vi "15-12-13 UHR-Fleezers Control (host) - 15.2.1UCB Darwin.vi"() -> ()   [LabVIEW 2014] (continued)
        n1238 = Select(t=w1811, s="+ phase (BI DO)", f="Phase adj. (BI DO)") -> (s? t:f=w1806:i16)
        n1239 = xnode "Read/Write Control"("FPGA VI Reference In"=w1803, "Phase count adjustment (GI)"=w1841, "Phase count adjustment (GI) 2"=w1829, "Phase count adjustment (RI)"=w1822, "Phase count adjustment (Green FB)"=w1817, "Phase count adjustment (BI AO)"=w1807, "Phase count adjustment (BI D)"=w1806) -> ("FPGA VI Reference Out"=w1839:T24, "error out"=w1840:errorcluster)  [unwired: 1 in]
        n1240 = xnode "Read/Write Control"("FPGA VI Reference In"=w1839, "error in"=w1840, "+ phase (GI)"=w1837, "+ phase (GI) 2"=w1828, "+ phase (RI)"=w1823, "+ phase (Green FB)"=w1816, "+ phase (BI AO)"=w1805, "+ phase (BI D)"=w1804) -> ("error out"=w1838:errorcluster)  [unwired: 1 out]
      }
      event "Green Laser ON/OFF", "Red Laser ON/OFF", "Blue Laser ON/OFF": Value Change {
        # "This loop shouldn't be initialized.  The main 'laser ON' settings should dominate and set the others."
        n1241 = event-data() -> ()  [unwired: 7 out]
        n1242 = property on="Red Laser ON" class="Bool (strict)"("Val(Sgnl)"="Red Laser ON/OFF") -> ()  [unwired: 2 in, 2 out]
        n1243 = property on="Blue Laser ON" class="Bool (strict)"("Val(Sgnl)"="Blue Laser ON/OFF") -> ()  [unwired: 2 in, 2 out]
        n1244 = property on="Green Laser ON" class="Bool (strict)"("Val(Sgnl)"="Green Laser ON/OFF") -> ()  [unwired: 2 in, 2 out]
      }
      event "Laser interlacing mode", "Green Laser ON", "Red Laser ON", "Blue Laser ON": Value Change {
        n1245 = event-data() -> ()  [unwired: 7 out]
        n1246 = local write "Green Laser ON/OFF"("Green Laser ON") -> ()
        n1247 = local write "Blue Laser ON/OFF"("Blue Laser ON") -> ()
        n1248 = local write "Red Laser ON/OFF"("Red Laser ON") -> ()
        n1249 = case shown="True" "Green Laser ON" {
          tunnel: "Laser interlacing mode" -> [_ w1903]
          tunnel: [enum32{"Laser ON", "Laser OFF", "Interlace"}."Laser OFF" ("Green laser mode") w1903] -> w1879
          tunnel: [FALSE w1899] -> w1878
          frame False {
          }
          frame True {
            n1250 = local read "Green FB On/Off"() -> (w1900:bool)
            n1251 = Equal?(x=w1903, y=enum32{"Laser ON", "Laser OFF", "Interlace"}."Interlace") -> (x = y?=w1901:bool)
            n1252 = And(x=w1901, y=w1900) -> (x .and. y?=w1899:bool)
          }
        }
        n1253 = case shown="True" "Red Laser ON" {
          tunnel: "Laser interlacing mode" -> [_ w1896]
          tunnel: [enum32{"Laser ON", "Laser OFF", "Interlace"}."Laser OFF" ("Green laser mode") w1896] -> w1875
          tunnel: [FALSE w1892] -> w1874
          frame False {
          }
          frame True {
            n1254 = local read "Red FB On/Off"() -> (w1893:bool)
            n1255 = Equal?(x=w1896, y=enum32{"Laser ON", "Laser OFF", "Interlace"}."Interlace") -> (x = y?=w1894:bool)
            n1256 = And(x=w1894, y=w1893) -> (x .and. y?=w1892:bool)
          }
        }
        n1257 = case shown="True" "Blue Laser ON" {
          tunnel: "Laser interlacing mode" -> [_ w1887]
          tunnel: [enum32{"Laser ON", "Laser OFF", "Interlace"}."Laser OFF" ("Green laser mode") w1887] -> w1871
          tunnel: [FALSE w1885] -> w1870
          frame False {
          }
          frame True {
            n1258 = local read "Blue FB On/Off"() -> (w1886:bool)
            n1259 = Equal?(x=w1887, y=enum32{"Laser ON", "Laser OFF", "Interlace"}."Interlace") -> (x = y?=w1888:bool)
            n1260 = And(x=w1888, y=w1886) -> (x .and. y?=w1885:bool)
          }
        }
        n1261 = xnode "Read/Write Control"("FPGA VI Reference In"=w1869, "Operating Mode"=w1879, "Operating Mode 2"=w1879, "Green FB On/Off"=w1878, "Red Laser Operating Mode"=w1875, "RI Operating Mode 2"=w1875, "Red FB On/Off"=w1874, "BI Operating Mode (AO)"=w1871, "Blue Laser Operating Mode (D)"=w1871, "Blue FB On/Off"=w1870) -> ("error out"=w1880:errorcluster)  [unwired: 1 in, 1 out]
        n1262 = local read "Red FB On/Off"() -> (w1852:bool)
        n1263 = local read "Green FB On/Off"() -> (w1854:bool)
        n1264 = local read "Green Laser ON"() -> (w1853:bool)
        n1265 = local read "Red Laser ON"() -> (w1851:bool)
        n1266 = And(x=w1852, y=w1851) -> (x .and. y?=w1857:bool)
        n1267 = And(x=w1854, y=w1853) -> (x .and. y?=w1863:bool)
        n1268 = local read "Red laser intensity (V)"() -> (w1856:dbl)
        n1269 = local read "Red FB Setpoint (mV)"() -> (w1855:dbl)
        n1270 = local read "Green FB Setpoint (mV)"() -> (w1866:dbl)
        n1271 = local read "Green laser intensity (V)"() -> (w1868:dbl)
        n1272 = Multiply(x=w1856, y=1000.0) -> (x*y=w1860:dbl)
        n1273 = Subtract(x=w1855, y=5.0) -> (x-y=w1859:dbl)
        n1274 = Multiply(x=w1868, y=1000.0) -> (x*y=w1865:dbl)
        n1275 = Subtract(x=w1866, y=5.0) -> (x-y=w1864:dbl)
        n1276 = Less Or Equal?(x=w1860, y=w1859) -> (x <= y?=w1858:bool)
        n1277 = Less Or Equal?(x=w1865, y=w1864) -> (x <= y?=w1862:bool)
        n1278 = And(x=w1857, y=w1858) -> (x .and. y?=w1847:bool)
        n1279 = And(x=w1863, y=w1862) -> (x .and. y?=w1848:bool)
        n1280 = Or(x=w1848, y=w1847) -> (x .or. y?=w1846:bool)
        n1281 = case shown="True" w1846 {
          frame False {
            n1282 = local write "Laser Intensity Low (bugs to fix)"(FALSE ("Laser Intensity Low")) -> ()
          }
          frame True {
            n1283 = local write "Laser Intensity Low (bugs to fix)"(TRUE ("Laser Intensity Low")) -> ()
          }
        }
      }
      event "Invert laser interlacing": Value Change {
        n1284 = event-data() -> ()  [unwired: 7 out]
        n1285 = xnode "Read/Write Control"("FPGA VI Reference In"=w1904, "Invert GI"="Invert laser interlacing", "Invert GI 2"="Invert laser interlacing", "Invert RI"="Invert laser interlacing", "Invert RI 2"="Invert laser interlacing", "Invert BI (AO)"="Invert laser interlacing", "Invert BI (D)"="Invert laser interlacing") -> ("error out"=w1906:errorcluster)  [unwired: 1 in, 1 out]
      }
      event "Green FB Setpoint (mV)", "Green FB Gains", "Green FB On/Off", "Green Intensity % (FB OFF)", "Green int current ON count adj": Value Change {
        n1286 = event-data() -> ()  [unwired: 7 out]
        n1287 = local read "Green FB Setpoint (mV)"() -> (w1926:dbl)
        n1288 = Multiply(x=w1926, y=3.2767) -> (x*y=w1925:dbl)
        n1289 = local read "Green Intensity % (FB OFF)"() -> (w1929:dbl)
        n1290 = Multiply(x=w1929, y=655.35) -> (x*y=w1930:dbl)
        n1291 = To Unsigned Word Integer(number=w1930) -> (unsigned 16bit integer=w1928:u16)
        n1292 = local read "Green int current ON count adj"() -> (w1932:u32)
        n1293 = local read "Laser interlacing mode"() -> (w1923:enum32{"Laser ON", "Laser OFF", "Interlace"})
        n1294 = local read "Green FB Gains"() -> (w1920:T11)
        n1295 = local read "Green Laser ON"() -> (w1924:bool)
        n1296 = local read "Green FB On/Off"() -> (w1933:bool)
        n1297 = Equal?(x=w1923, y=enum32{"Laser ON", "Laser OFF", "Interlace"}."Interlace") -> (x = y?=w1921:bool)
        n1298 = Unbundle By Name(w1920) -> ("proportional gain (Kc)"=w1919:i16, "integral gain (Kc*Ts/Ti)"=w1918:i16, "derivative gain (Kc*Td/Ts)"=w1917:i16)
        n1299 = Compound Arithmetic op=AND(w1921, w1933, w1924) -> (w1907:bool)
        n1300 = local read "Green FB Setpoint (mV)"() -> (w1911:dbl)
        n1301 = local read "Green laser intensity (V)"() -> (w1914:dbl)
        n1302 = xnode "Read/Write Control"("FPGA VI Reference In"=w1916, "Green FB Setpoint"=w1925, "Green FB On/Off"=w1907, "Current Out"=w1928, "Green int current ON count adj"=w1932, "P3"=w1919, "I3"=w1918, "D3"=w1917) -> ("error out"=w1934:errorcluster)  [unwired: 1 in, 1 out]
        n1303 = Multiply(x=w1914, y=1000.0) -> (x*y=w1910:dbl)
        n1304 = Subtract(x=w1911, y=5.0) -> (x-y=w1909:dbl)
        n1305 = Less Or Equal?(x=w1910, y=w1909) -> (x <= y?=w1908:bool)
        n1306 = And(x=w1907, y=w1908) -> (x .and. y?=w1915:bool)
        n1307 = case shown="True" w1915 {
          frame False {
            n1308 = local write "Laser Intensity Low (bugs to fix)"(FALSE ("Laser Intensity Low")) -> ()
          }
          frame True {
            n1309 = local write "Laser Intensity Low (bugs to fix)"(TRUE ("Laser Intensity Low")) -> ()
          }
        }
      }
      event "Blue FB Setpoint (mV)", "Blue FB Gains", "Blue FB On/Off", "Blue Intensity % (FB OFF)", "Blue int AO ON count adjust": Value Change {
        # "Triggers blue laser serial command"
        # "16 bit analog out"
        n1310 = event-data() -> ()  [unwired: 7 out]
        n1311 = Multiply(x="Blue FB Setpoint (mV)", y=3.2767) -> (x*y=w1954:dbl)
        n1312 = Multiply(x="Blue Intensity % (FB OFF)", y=0.8) -> (x*y=w1937:dbl)
        n1313 = Number To Decimal String(number=w1937) -> (decimal integer string=w1938:string)  [unwired: 1 in]
        n1314 = Multiply(x="Blue Intensity % (FB OFF)", y=655.35) -> (x*y=w1957:dbl)
        n1315 = local write "Blue Laser Power (mW)\n(Constant Power Mode)"(w1938) -> ()
        n1316 = To Unsigned Word Integer(number=w1957) -> (unsigned 16bit integer=w1956:u16)
        n1317 = local read "Laser interlacing mode"() -> (w1952:enum32{"Laser ON", "Laser OFF", "Interlace"})
        n1318 = Unbundle By Name("Blue FB Gains") -> ("proportional gain (Kc)"=w1949:i16, "integral gain (Kc*Ts/Ti)"=w1948:i16, "derivative gain (Kc*Td/Ts)"=w1947:i16)
        n1319 = local read "Blue Laser ON"() -> (w1942:bool)
        n1320 = Equal?(x=w1952, y=enum32{"Laser ON", "Laser OFF", "Interlace"}."Interlace") -> (x = y?=w1950:bool)
        n1321 = Compound Arithmetic op=AND(w1950, "Blue FB On/Off", w1942) -> (w1953:bool)
        n1322 = xnode "Read/Write Control"("FPGA VI Reference In"=w1941, "Blue FB Setpoint"=w1954, "Blue FB On/Off"=w1953, "BI Current Out"=w1956, "Blue current ON count adj (AO)"="Blue int AO ON count adjust", "P5"=w1949, "I5"=w1948, "D5"=w1947) -> ("error out"=w1959:errorcluster)  [unwired: 1 in, 1 out]
      }
      event "Red FB Setpoint (mV)", "Red FB Gains", "Red FB On/Off", "Red Intensity % (FB OFF)": Value Change {
        n1323 = event-data() -> ()  [unwired: 7 out]
        n1324 = local read "Red FB Setpoint (mV)"() -> (w1980:dbl)
        n1325 = Multiply(x=w1980, y=3.2767) -> (x*y=w1979:dbl)
        n1326 = local read "Red Intensity % (FB OFF)"() -> (w1970:dbl)
        n1327 = Multiply(x=w1970, y=655.35) -> (x*y=w1983:dbl)
        n1328 = To Unsigned Word Integer(number=w1983) -> (unsigned 16bit integer=w1982:u16)
        n1329 = local read "Laser interlacing mode"() -> (w1977:enum32{"Laser ON", "Laser OFF", "Interlace"})
        n1330 = local read "Red FB Gains"() -> (w1974:T11)
        n1331 = local read "Red Laser ON"() -> (w1978:bool)
        n1332 = local read "Red FB On/Off"() -> (w1985:bool)
        n1333 = Equal?(x=w1977, y=enum32{"Laser ON", "Laser OFF", "Interlace"}."Interlace") -> (x = y?=w1975:bool)
        n1334 = Unbundle By Name(w1974) -> ("proportional gain (Kc)"=w1973:i16, "integral gain (Kc*Ts/Ti)"=w1972:i16, "derivative gain (Kc*Td/Ts)"=w1971:i16)
        n1335 = Compound Arithmetic op=AND(w1975, w1985, w1978) -> (w1962:bool)
        n1336 = local read "Red laser intensity (V)"() -> (w1961:dbl)
        n1337 = local read "Red FB Setpoint (mV)"() -> (w1960:dbl)
        n1338 = xnode "Read/Write Control"("FPGA VI Reference In"=w1969, "Red FB Setpoint"=w1979, "Red FB On/Off"=w1962, "RI Current Out"=w1982, "P4"=w1973, "I4"=w1972, "D4"=w1971) -> ("error out"=w1986:errorcluster)  [unwired: 1 in, 1 out]
        n1339 = Multiply(x=w1961, y=1000.0) -> (x*y=w1966:dbl)
        n1340 = Subtract(x=w1960, y=5.0) -> (x-y=w1965:dbl)
        n1341 = Less Or Equal?(x=w1966, y=w1965) -> (x <= y?=w1964:bool)
        n1342 = And(x=w1962, y=w1964) -> (x .and. y?=w1963:bool)
        n1343 = case shown="False" w1963 {
          frame False {
            n1344 = local write "Laser Intensity Low (bugs to fix)"(FALSE ("Laser Intensity Low")) -> ()
          }
          frame True {
            n1345 = local write "Laser Intensity Low (bugs to fix)"(TRUE ("Laser Intensity Low")) -> ()
          }
        }
      }
      event "+ phase (APD 1 Gate)", "- phase (APD 1 Gate)", "+ phase (APD 2 Gate)", "- phase (APD 2 Gate)", "+ phase (APD 3 Gate)", "- phase (APD 3 Gate)", "+ phase (APD Acq)", "- phase (APD Acq)": Value Change {
        n1346 = event-data() -> ()  [unwired: 7 out]
        n1347 = local read "Phase Adj. (APD 1 Gate)"() -> (w2009:i16)
        n1348 = Or(x="- phase (APD 1 Gate)", y="+ phase (APD 1 Gate)") -> (x .or. y?=w2011:bool)
        n1349 = Negate(x=w2009) -> (-x=w2016:i16)
        n1350 = Select(t=w2016, s="+ phase (APD 1 Gate)", f=w2009) -> (s? t:f=w2015:i16)
        n1351 = local read "Phase Adj. (APD 2 Gate)"() -> (w2006:i16)
        n1352 = Or(x="- phase (APD 2 Gate)", y="+ phase (APD 2 Gate)") -> (x .or. y?=w2004:bool)
        n1353 = Negate(x=w2006) -> (-x=w2008:i16)
        n1354 = Select(t=w2008, s="+ phase (APD 2 Gate)", f=w2006) -> (s? t:f=w2005:i16)
        n1355 = Negate(x="Phase Adj. (APD 3 Gate)") -> (-x=w2003:i16)
        n1356 = Or(x="- phase (APD 3 Gate)", y="+ phase (APD 3 Gate)") -> (x .or. y?=w1999:bool)
        n1357 = Select(t=w2003, s="+ phase (APD 3 Gate)", f="Phase Adj. (APD 3 Gate)") -> (s? t:f=w2000:i16)
        n1358 = local read "Phase Adj. (APD Acq)"() -> (w1997:i16)
        n1359 = Or(x="- phase (APD Acq)", y="+ phase (APD Acq)") -> (x .or. y?=w1995:bool)
        n1360 = Negate(x=w1997) -> (-x=w1998:i16)
        n1361 = Select(t=w1998, s="+ phase (APD Acq)", f=w1997) -> (s? t:f=w1996:i16)
        n1362 = xnode "Read/Write Control"("FPGA VI Reference In"=w1989, "Phase count adjustment (APD 1 Gate)"=w2015, "Phase count adjustment (APD 2 Gate)"=w2005, "Phase count adjustment (APD 3 Gate)"=w2000, "Phase Count Adjustment (APD Acq)"=w1996) -> ("FPGA VI Reference Out"=w2013:T24, "error out"=w2014:errorcluster)  [unwired: 1 in]
        n1363 = xnode "Read/Write Control"("FPGA VI Reference In"=w2013, "error in"=w2014, "+ phase (APD 1 Gate)"=w2011, "+ phase (APD 2 Gate)"=w2004, "+ phase (APD 3 Gate)"=w1999, "+ phase (APD Acq)"=w1995) -> ("error out"=w2012:errorcluster)  [unwired: 1 out]
      }
      event "Invert APD Gate", "APD Gate ON Count", "APD Gate OFF Count", "APD Gate", "APD Integration Time (s)", "APD AO Scale Factor", "Duty Frequency (ON 1/N cycles)", "Interlace ON count", "Interlace OFF count": Value Change {
        n1364 = event-data() -> ()  [unwired: 7 out]
        n1365 = Add(x="Interlace ON count", y="Interlace OFF count") -> (x+y=w2023:u16)
        n1366 = Add(x="APD Gate ON Count", y="APD Gate OFF Count") -> (x+y=w2034:u16)
        n1367 = Multiply(x="Duty Frequency (ON 1/N cycles)", y=w2023) -> (x*y=w2019:u16)
        "Green AI Count" <- w2019
        "Red AI Count" <- w2019
        "Blue AI Count" <- w2019
        n1368 = Subtract(x=w2019, y="Interlace ON count") -> (x-y=w2022:u16)
        n1369 = Multiply(x=w2034, y="Duty Frequency (ON 1/N cycles)") -> (x*y=w2033:u16)
        n1370 = Subtract(x=w2033, y="APD Gate ON Count") -> (x-y=w2032:u16)
        n1371 = local read "DMA Update Period (s)"() -> (w2035:dbl)
        n1372 = Multiply(x="APD Integration Time (s)", y=40000000.0) -> (x*y=w2039:dbl)
        n1373 = Reciprocal(x="APD Integration Time (s)") -> (1/x=→"APD Acq Rate (Hz)":dbl)
        n1374 = To Unsigned Long Integer(number=w2039) -> (unsigned 32bit integer=w2025:u32)
        "APD Int. Count" <- w2025
        n1375 = local read "Number of APDs"() -> (w2018:u8)
        n1376 = Divide(x=w2035, y="APD Integration Time (s)") -> (x/y=w2037:dbl)
        n1377 = Multiply(x=w2018, y=w2037) -> (x*y=w2036:dbl)
        n1378 = local write "APD Samples/FIFO Acq."(w2037) -> ()
        n1379 = local write "APD Elements/DMA read"(w2036) -> ()
        n1380 = xnode "Read/Write Control"("FPGA VI Reference In"=w2017, "Invert APD Gate"="Invert APD Gate", "APD Gate ON Count"="APD Gate ON Count", "APD Gate OFF Count"=w2032, "APD Acq Rate Count"=w2025, "APD Gate Operating Mode"="APD Gate", "APD AO scale factor"="APD AO Scale Factor", "Green interlace ON count"="Interlace ON count", "Green interlace OFF count"=w2022, "Green interlace ON count 2"="Interlace ON count", "Green interlace OFF count 2"=w2022, "Green FB Count"=w2019, "Red interlace ON count"="Interlace ON count", "Red interlace OFF count"="Interlace OFF count", "Blue ON count (AO)"="Interlace ON count", "Blue OFF count (AO)"="Interlace OFF count", "Blue interlace OFF count (D)"="Interlace OFF count", "Blue interlace ON count (D)"="Interlace ON count") -> ("error out"=w2041:errorcluster)  [unwired: 1 in, 1 out]
      }
      event "Neg. TTrig FPGA": Value Change {
        n1381 = event-data() -> ()  [unwired: 7 out]
        n1382 = xnode "Read/Write Control"("FPGA VI Reference In"=w2042, "TTrig Negate Pos"="Neg. TTrig FPGA") -> ()  [unwired: 1 in, 2 out]
      }
      event "Test ttrig": Value Change {
        n1383 = event-data() -> ()  [unwired: 7 out]
        n1384 = xnode "Read/Write Control"("FPGA VI Reference In"=w2044, "TTrig?"=TRUE) -> ("error out"=w2046:errorcluster)  [unwired: 1 in, 1 out]
      }
      event "Number of F/B Scans (AOD)", "Scan Speed (nm/s)", "Scan BD", "Initial delta (MHz)", "Step Size (nm)", "Scan Range (nm)": Value Change {
        w2110 = 123.0  # AOM cal (nm/MHz)
        n1385 = event-data() -> ()  [unwired: 7 out]
        n1386 = local read "BD 1 Frequency 1 (MHz)"() -> (w2093:dbl)
        n1387 = local read "AOM X Cal (nm/MHz)"() -> (w2085:dbl)
        n1388 = local read "X RF Frequency Limits (MHz)"() -> (w2097:T18)
        n1389 = local read "Y RF Frequency Limits (MHz)"() -> (w2094:T18)
        n1390 = local read "BD 2 Frequency 1 (MHz)"() -> (w2099:dbl)
        n1391 = Negate(x="Scan Range (nm)") -> (-x=w2063:dbl)
        n1392 = Divide(x=w2063, y=w2085) -> (x/y=w2067:dbl)
        n1393 = Select(t=w2097, s="Scan BD", f=w2094) -> (s? t:f=w2096:T18)
        n1394 = Select(t=w2093, s="Scan BD", f=w2099) -> (s? t:f=w2098:dbl)
        n1395 = Unbundle By Name(w2096) -> ("Maximum"=w2105:dbl, "Minimum"=w2104:dbl)
        n1396 = Add(x=w2067, y=w2098) -> (x+y=w2102:dbl)
        n1397 = Divide(x=w2063, y="Step Size (nm)") -> (x/y=w2082:dbl)
        n1398 = Divide(x="Step Size (nm)", y=w2085) -> (x/y=w2091:dbl)
        n1399 = Absolute Value(x=w2082) -> (abs(x)=w2066:dbl)
        n1400 = Sign(1:w2063) -> (0:w2064:dbl)
        n1401 = In Range and Coerce(upper limit=w2105, x=w2102, lower limit=w2104) -> (coerced(x)=w2101:dbl, In Range?=w2103:bool)
        n1402 = To Unsigned Quad Integer(1:w2066) -> (0:w2081:u64)
        "Scan steps (AOD)" <- w2081
        n1403 = call "IR AOM freq to word.vi"("Frequency In (MHz)"=w2091) -> ("Frequency Word Out (double)"=w2088:dbl)
        n1404 = Multiply(x=w2064, y=w2088) -> (x*y=w2065:dbl)
        n1405 = Subtract(x=w2102, y=w2101) -> (x-y=w2100:dbl)
        n1406 = To Quad Integer(1:w2065) -> (0:w2087:i64)
        "Incr. int (AOD)" <- w2087
        n1407 = Subtract(x=w2067, y=w2100) -> (x-y=w2086:dbl)
        "Scan Range (MHz)" <- w2086
        n1408 = Select(t=w2067, s=w2103, f=w2086) -> (s? t:f=w2106:dbl)
        n1409 = Multiply(x=w2086, y=w2085) -> (x*y=w2084:dbl)
        n1410 = Decrement(x=w2081) -> (x-1=w2134:u64)
        n1411 = Negate(x=w2084) -> (-x=w2080:dbl)
        n1412 = local write "Scan Range (nm)"(w2080) -> ()
        n1413 = Divide(x=w2106, y=w2134) -> (x/y=w2090:dbl)
        "Scan Increment (MHz)" <- w2090
        n1414 = call "IR AOM freq to word.vi"("Frequency In (MHz)"=w2090) -> ("Frequency Word Out (double)"=w2089:dbl)
        n1415 = Divide(x="Step Size (nm)", y="Scan Speed (nm/s)") -> (x/y=w2077:dbl)
        n1416 = To Quad Integer(1:w2089) -> ()  [unwired: 1 out]
        n1417 = local read "Number Interlace Sets"() -> (w2061:u8)
        n1418 = local read "AI Count (ticks)"() -> (w2062:u16)
        n1419 = local read "Total Counts (ticks)"() -> (w2060:u16)
        n1420 = local read "# Samples/trap"() -> (w2092:u32)
        n1421 = Multiply(x=w2062, y=w2061) -> (x*y=w2059:u16)
        n1422 = Divide(x=w2060, y=w2059) -> (x/y=w2058:dbl)
        n1423 = Select(t=w2093, s="Scan BD", f=w2099) -> (s? t:f=w2131:dbl)
        "Initial freq. (MHz)" <- w2131
        n1424 = Add(x=w2106, y=w2131) -> (x+y=→"Final freq. (MHz)":dbl)
        n1425 = Divide(x=w2060, y=40000000.0) -> (x/y=w2076:dbl)
        n1426 = Divide(x=w2077, y=w2076) -> (x/y=w2075:dbl)
        n1427 = To Unsigned Quad Integer(1:w2075) -> (0:w2050:u64)
        n1428 = Quotient & Remainder(x=w2050, y=u64 2) -> (x-y*floor(x/y)=w2054:u64)  [unwired: 1 out]
        n1429 = Equal?(x=w2054, y=u64 0) -> (x = y?=w2052:bool)
        n1430 = Decrement(x=w2050) -> (x-1=w2051:u64)
        n1431 = Select(t=w2050, s=w2052, f=w2051) -> (s? t:f=w2049:u64)
        "Cycles/step (AOD)" <- w2049
        n1432 = xnode "Read/Write Control"("FPGA VI Reference In"=w2048, "Scan steps"=w2081, "Number of scans"="Number of F/B Scans (AOD)", "Cycles per step"=w2049, "Scan freq.  increment"=w2087, "Scan BD"="Scan BD") -> ("error out"=w2140:errorcluster)  [unwired: 1 in, 1 out]
        n1433 = Multiply(x=w2081, y=w2049) -> (x*y=w2135:u64)
        n1434 = Multiply(x=w2135, y=u64 2) -> (x*y=w2057:u64)
        n1435 = Multiply(x=w2058, y=w2057) -> (x*y=w2056:dbl)
        "Data points/scan (f/b)" <- w2056
        n1436 = Multiply(x=w2056, y="Number of F/B Scans (AOD)") -> (x*y=w2138:dbl)
        "Data points/scans" <- w2138
        n1437 = Divide(x=w2138, y=w2092) -> (x/y=→"N sets should be saved":dbl)
        n1438 = Multiply(x=w2135, y=w2076) -> (x*y=w2074:dbl)
        "Time/Scan (s) (AOD)" <- w2074
        n1439 = Select(t=w2106, s="Scan BD", f=0.0) -> (s? t:f=w2132:dbl)
        n1440 = Select(t=0.0, s="Scan BD", f=w2106) -> (s? t:f=w2128:dbl)
        n1441 = local read "BD 2 Frequency 2 (MHz)"() -> (w2124:dbl)
        n1442 = local read "BD 1 Frequency 2 (MHz)"() -> (w2127:dbl)
        n1443 = Add(x=w2128, y=w2099) -> (x+y=w2125:dbl)
        n1444 = Add(x=w2093, y=w2132) -> (x+y=w2126:dbl)
        n1445 = Multiply(x=w2074, y=2.0) -> (x*y=w2073:dbl)
        n1446 = Multiply(x=w2073, y="Number of F/B Scans (AOD)") -> (x*y=w2070:dbl)
        n1447 = Divide(x=w2070, y=60.0) -> (x/y=→"Time to Finish All (min)":dbl)
        n1448 = Add(x="Trap 2 Bead Size (nm)", y="Trap 1 Bead Size (nm)") -> (x+y=w2114:dbl)
        n1449 = Divide(x=w2114, y=2.0) -> (x/y=w2108:dbl)
        n1450 = local read "Initial delta (MHz)"() -> (w2111:dbl)
        n1451 = Subtract(x=w2125, y=w2124) -> (x-y=w2122:dbl)
        n1452 = Subtract(x=w2126, y=w2127) -> (x-y=w2123:dbl)
        n1453 = Square(x=w2122) -> (x^2=w2121:dbl)
        n1454 = Square(x=w2123) -> (x^2=w2120:dbl)
        n1455 = Add(x=w2120, y=w2121) -> (x+y=w2119:dbl)
        n1456 = Square Root(x=w2119) -> (sqrt(x)=w2118:dbl)
        "Final delta (MHz)" <- w2118
        n1457 = Multiply(x=w2110, y=w2118) -> (x*y=w2117:dbl)
        n1458 = Multiply(x=w2111, y=w2110) -> (x*y=w2109:dbl)
        n1459 = Subtract(x=w2109, y=w2108) -> (x-y=→"Initial sep (nm)":dbl)
        n1460 = Subtract(x=w2117, y=w2108) -> (x-y=→"Final sep (nm)":dbl)
      }
      event "Freq or Amp switch first", "Swap F1 and F2", "Freq switch delay", "Amp switch delay": Value Change {
        n1461 = event-data() -> ()  [unwired: 7 out]
        n1462 = local read "Amp switch delay"() -> (w2142:u16)
        n1463 = local read "Swap F1 and F2"() -> (w2143:bool)
        n1464 = xnode "Read/Write Control"("FPGA VI Reference In"=w2141, "Swap F1 and F2"=w2143, "Amp switch delay"=w2142) -> ("error out"=w2144:errorcluster)  [unwired: 1 in, 1 out]
      }
      event "Scan steps (MCL)", "Number of scans (MCL)", "Scan Range (V)\n(of steps)", "2D or 1D Scan", "N APD Samp/step", "Fast Scan Dir", "Continuous MCL Scanning", "Scan lines (y)": Value Change {
        w2147 = 32767.0 ("y")
        n1465 = event-data() -> ()  [unwired: 7 out]
        n1466 = Select(t="Scan lines (y)", s="2D or 1D Scan", f="Number of scans (MCL)") -> (s? t:f=w2152:u64)
        n1467 = Decrement(x="Scan steps (MCL)") -> (x-1=w2168:u64)
        n1468 = Divide(x="Scan Range (V)\n(of steps)", y=w2168) -> (x/y=w2167:dbl)
        "Desired Scan Incr (V)" <- w2167
        n1469 = local read "APD Integration Time (s)"() -> (w2160:dbl)
        n1470 = Multiply(x=w2167, y=w2147) -> (x*y=w2176:dbl)
        n1471 = Divide(x=w2176, y=10.0) -> (x/y=w2166:dbl)
        "Desired incr (int)" <- w2166
        n1472 = local read "Update Count (MCL)"() -> (w2172:u32)
        n1473 = Round Toward -Infinity(1:w2166) -> (0:w2175:dbl)
        n1474 = To Word Integer(number=w2175) -> (16bit integer=w2150:i16)
        "Actual Incr. int (MCL)" <- w2150
        n1475 = Multiply(x=w2160, y=40000000.0) -> (x*y=w2173:dbl)
        n1476 = Divide(x=w2173, y=w2172) -> (x/y=w2171:dbl)
        n1477 = Multiply(x=i16 10, y=w2150) -> (x*y=w2148:i16)
        n1478 = Multiply(x="N APD Samp/step", y=w2171) -> (x*y=w2170:dbl)
        "Cycles/step (MCL)" <- w2170
        n1479 = Divide(x=w2148, y=w2147) -> (x/y=→"Actual MCL Inc (V)":dbl)
        n1480 = Multiply(x="N APD Samp/step", y="Scan steps (MCL)") -> (x*y=w2162:dbl)
        n1481 = local read "APD Samples/FIFO Acq."() -> (w2159:dbl)
        n1482 = Multiply(x=w2162, y=u64 2) -> (x*y=w2161:dbl)
        "Data points/scan (f+b)" <- w2161
        n1483 = Multiply(x=w2161, y=w2152) -> (x*y=w2179:dbl)
        "Data points/scans (MCL)" <- w2179
        n1484 = Multiply(x=w2160, y=w2161) -> (x*y=w2153:dbl)
        "Time/f+b scan (s) (MCL)" <- w2153
        n1485 = Divide(x=w2179, y=w2159) -> (x/y=→"N sets should be saved (MCL)":dbl)
        n1486 = Multiply(x=w2153, y=w2152) -> (x*y=→"Total Time (s)":dbl)
        n1487 = Not(x="Fast Scan Dir") -> (.not. x?=w2157:bool)
        n1488 = xnode "Read/Write Control"("FPGA VI Reference In"=w2145, "Scan steps (MCL)"="Scan steps (MCL)", "Number of scans (MCL)"=w2152, "Cycles per step (MCL)"=w2170, "Scan freq.  increment (MCL)"=w2150, "1D or 2D Scan?"="2D or 1D Scan", "MCL Scan Axis"=w2157, "Cont. Scan (MCL)"="Continuous MCL Scanning") -> ("error out"=w2181:errorcluster)  [unwired: 1 in, 1 out]
      }
      event "Read Cal": Value Change {
        w2193 = 1000.0 ("y")
        n1489 = event-data() -> ()  [unwired: 7 out]
        n1490 = local read "Save file name"() -> (w2212:path)
        n1491 = local write "Read Cal"(FALSE ("Read Cal")) -> ()
        n1492 = Strip Path(path=w2212) -> (stripped path=w2211:path)  [unwired: 1 out]
        n1493 = Path To String(path=w2211) -> (string=w2210:string)
        n1494 = Concatenate Strings(w2210, "\\current.cal" ("string")) -> (w2208:string)
        n1495 = String To Path(string=w2208) -> (path=w2207:path)
        n1496 = Open/Create/Replace File(file path (use dialog)=w2207, operation (0:open)=T33."open", access (0:read/write)=enum16{"read/write", "read-only", "write-only"}."read-only") -> (refnum out=w2215:refnum<file>, error out=w2201:errorcluster)  [unwired: 1 in, 3 out]
        n1497 = Deny Access(4:w2201, 7:w2215) -> (0:w2200:errorcluster, 3:w2206:refnum<file>)  [unwired: 1 out]
        n1498 = Read from Binary File(5:0.0, 8:w2200, 9:T32."big-endian, network order" ("byte order (0:big-endian, network order)"), 10:-1 ("count (1)"), 11:w2206) -> (0:w2199:errorcluster, 2:w2197:dbl[], 3:w2202:refnum<file>)  [unwired: 2 out]
        n1499 = Array To Cluster(array=w2197) -> (cluster=w2196:T35)
        n1500 = Unbundle(w2196) -> ("[0]"=w2190:dbl, "[1]"=w2184:dbl, "[2]"=w2188:dbl, "[3]"=w2182:dbl, "[4]"=w2195:dbl, "[5]"=w2194:dbl)
        n1501 = Close File(refnum=w2202, error in=w2199) -> (error out=→"Read cal error":errorcluster)  [unwired: 1 out]
        n1502 = Multiply(x=w2195, y=w2193) -> (x*y=w2189:dbl)
        n1503 = Multiply(x=w2194, y=w2193) -> (x*y=w2183:dbl)
        n1504 = Bundle By Name(cluster="T1 calibration", "T1 alpha_x (nm/V)"=w2190, "T1 offset_x (mV)"=w2189, "T1 kappa_x (pN/nm)"=w2188) -> (w2187:T6)
        n1505 = Bundle By Name(cluster="T2 calibration", "T2 alpha_x (nm/V)"=w2184, "T2 offset_x (mV)"=w2183, "T2 kappa_x (pN/nm)"=w2182) -> (w2185:T5)
        n1506 = local write "T1 calibration"(w2187) -> ()
        n1507 = local write "T2 calibration"(w2185) -> ()
      }
      event "Abort MCL Scan": Value Change {
        n1508 = event-data() -> ()  [unwired: 7 out]
        n1509 = local write "MCL Scanning"(FALSE ("MCL Scanning")) -> ()
        n1510 = xnode "Read/Write Control"("FPGA VI Reference In"=w2216, "Abort scan (MCL)"="Abort MCL Scan") -> ("error out"=w2219:errorcluster)  [unwired: 1 in, 1 out]
      }
      event "Update Count (MCL)": Value Change {
        n1511 = event-data() -> ()  [unwired: 7 out]
        n1512 = xnode "Read/Write Control"("FPGA VI Reference In"=w2220, "MCL count"="Update Count (MCL)") -> ("error out"=w2222:errorcluster)  [unwired: 1 in, 1 out]
      }
      event "+ phase (MCL)", "- phase (MCL)": Value Change {
        n1513 = event-data() -> ()  [unwired: 7 out]
        n1514 = Or(x="- phase (MCL)", y="+ phase (MCL)") -> (x .or. y?=w2226:bool)
        n1515 = Negate(x="Phase adjust (MCL)") -> (-x=w2232:i16)
        n1516 = Select(t=w2232, s="+ phase (MCL)", f="Phase adjust (MCL)") -> (s? t:f=w2230:i16)
        n1517 = xnode "Read/Write Control"("FPGA VI Reference In"=w2223, "Phase count adjustment (MCL)"=w2230) -> ("FPGA VI Reference Out"=w2227:T24, "error out"=w2228:errorcluster)  [unwired: 1 in]
        n1518 = xnode "Read/Write Control"("FPGA VI Reference In"=w2227, "error in"=w2228, "+ phase (MCL)"=w2226) -> ("error out"=w2225:errorcluster)  [unwired: 1 out]
      }
      event "Abort AOD Scan": Value Change {
        n1519 = event-data() -> ()  [unwired: 7 out]
        n1520 = xnode "Read/Write Control"("FPGA VI Reference In"=w2233, "Abort scan"="Abort AOD Scan") -> ("error out"=w2235:errorcluster)  [unwired: 1 in, 1 out]
      }
      event "Continuous AOD Scanning": Value Change {
        n1521 = event-data() -> ()  [unwired: 7 out]
        n1522 = xnode "Read/Write Control"("FPGA VI Reference In"=w2236, "Cont. Scan"="Continuous AOD Scanning") -> ("error out"=w2238:errorcluster)  [unwired: 1 in, 1 out]
      }
      event "Index": Value Change {
        n1523 = event-data() -> ()  [unwired: 7 out]
        n1524 = call "Create new save file.vi"("Insert"="", "Ext"=".dat" ("string"), "Index In"="Index") -> ("Path Out"=→"Save file name":path, "Index Out"=w2239:dbl)
        "Save index" <- w2239
        n1525 = local write "Index"(w2239) -> ()
      }
      event "AO1", "AO2": Value Change {
        w2253 = 10.0 ("y")
        w2252 = 32767.0 ("y")
        n1526 = event-data() -> ()  [unwired: 7 out]
        n1527 = local read "AO2"() -> (w2251:dbl)
        n1528 = local read "AO1"() -> (w2248:dbl)
        n1529 = Multiply(x=w2248, y=w2252) -> (x*y=w2247:dbl)
        n1530 = Multiply(x=w2251, y=w2252) -> (x*y=w2250:dbl)
        n1531 = Divide(x=w2247, y=w2253) -> (x/y=w2246:dbl)
        n1532 = Divide(x=w2250, y=w2253) -> (x/y=w2249:dbl)
        n1533 = To Word Integer(number=w2246) -> (16bit integer=w2254:i16)
        n1534 = To Word Integer(number=w2249) -> (16bit integer=w2255:i16)
        n1535 = xnode "Read/Write Control"("FPGA VI Reference In"=w2244, "AO1"=w2254, "AO2"=w2255) -> ("error out"=w2245:errorcluster)  [unwired: 1 in, 1 out]
      }
      event "Inject Pump 1": Value Change {
        n1536 = event-data() -> ()  [unwired: 7 out]
        n1537 = local read "Use Harvard pumps\nfor beads (else Chemyx)"() -> (w2257:bool)
        n1538 = case shown="True" w2257 {
          tunnel: "Inject Pump 1" -> [w2261 w2302]
          tunnel: w2256 -> [_ w2303]
          frame False {
            n1539 = local read "Pump write delay (ms)"() -> (w2260:dbl)
            n1540 = local read "Chemyx Syringe Pump Serial Port"() -> (w2259:refnum<visa-resource-name>)
            n1541 = case shown="True" w2261 {
              tunnel: w2260 -> [w2267 w2281]
              tunnel: w2259 -> [w2264 w2280]
              frame False {
                n1542 = flat-sequence {
                  tunnel: w2264 -> [w2268]
                  tunnel: [w2268] -> w2265
                  tunnel: w2267 -> [_]
                  tunnel: [w2271] -> w2266
                  tunnel: w2265 -> [w2271]
                  tunnel: w2266 -> [w2272]
                  tunnel: [w2272] -> w2262
                  tunnel: [w2274] -> w2263
                  tunnel: w2262 -> [w2274]
                  tunnel: w2263 -> [w2276]
                  frame #0 {
                    n1543 = call "Write to pump.vi"("string"="enter pump1", "VISA resource name"=w2268) -> ()  [unwired: 1 out]
                  }
                  frame #1 {
                    n1544 = Wait (ms)(milliseconds to wait="Pump pause delay (ms)") -> ()  [unwired: 1 out]
                  }
                  frame #2 {
                    n1545 = call "Write to pump.vi"("string"="stop", "VISA resource name"=w2272) -> ()  [unwired: 1 out]
                  }
                  frame #3 {
                    n1546 = Wait (ms)(milliseconds to wait=u32 500) -> ()  [unwired: 1 out]
                  }
                  frame #4 {
                    n1547 = call "Write to pump.vi"("string"="stop", "VISA resource name"=w2276) -> ()  [unwired: 1 out]
                  }
                }
              }
              frame True {
                n1548 = flat-sequence {
                  tunnel: w2280 -> [w2290]
                  tunnel: w2281 -> [w2285]
                  tunnel: w2281 -> [w2292]
                  tunnel: w2280 -> [w2293]
                  tunnel: [w2293] -> w2278
                  tunnel: [w2295] -> w2279
                  tunnel: w2278 -> [w2295]
                  tunnel: w2279 -> [w2297]
                  frame #0 {
                    n1549 = local read "All Pump Parameters"() -> (w2284:T7)
                    n1550 = Unbundle By Name(w2284) -> ("Pump 1"=w2291:T36)
                    n1551 = call "Set pump parameters.vi"("Pump write delay (ms)"=w2285, "Volume (uL)"="Ch 1 Inject Volume (uL)", "Rate (uL/h)"="Ch 1 Inject Rate (ul/h)", "Units"=4.0, "Pump #"=1.0, "Pump Parameters In"=w2291, "VISA resource name"=w2290) -> ("Pump Parameters Out"=w2283:T36)  [unwired: 3 in]
                    n1552 = Bundle By Name(cluster=w2284, "Pump 1"=w2283) -> (w2282:T7)
                    n1553 = local write "All Pump Parameters"(w2282) -> ()
                  }
                  frame #1 {
                    n1554 = Wait (ms)(milliseconds to wait=w2292) -> ()  [unwired: 1 out]
                  }
                  frame #2 {
                    n1555 = call "Write to pump.vi"("string"="start", "VISA resource name"=w2293) -> ()  [unwired: 1 out]
                  }
                  frame #3 {
                    n1556 = Wait (ms)(milliseconds to wait=u32 500) -> ()  [unwired: 1 out]
                  }
                  frame #4 {
                    n1557 = call "Write to pump.vi"("string"="start", "VISA resource name"=w2297) -> ()  [unwired: 1 out]
                  }
                }
              }
            }
          }
          frame True {
            n1558 = case shown="False" w2302 {
              tunnel: w2303 -> [w2315 w2325]
              frame False {
                n1559 = flat-sequence {
                  tunnel: w2315 -> [w2317]
                  frame #0 {
                    n1560 = local write "Flushing P1"(FALSE ("Flushing P1")) -> ()
                    n1561 = Concatenate Strings("stop" ("string"), "\r") -> (w2319:string)
                    n1562 = VISA Write(VISA resource name=w2317, write buffer=w2319) -> ()  [unwired: 1 in, 3 out]
                  }
                  frame #1 {
                    n1563 = property on="Clear Volume P1" class="Bool (strict)"("Val(Sgnl)"=TRUE ("Value (Signaling)")) -> ()  [unwired: 2 in, 2 out]
                  }
                }
              }
              frame True {
                n1564 = local read "Normal Flow Rate (ul/h) P1"() -> (w2323:dbl)
                n1565 = Number To Decimal String(number=w2323) -> (decimal integer string=w2329:string)  [unwired: 1 in]
                n1566 = Concatenate Strings("irate  " ("string"), w2329, " u/h" ("string"), "\r") -> (w2327:string)
                n1567 = VISA Write(VISA resource name=w2325, write buffer=w2327) -> (VISA resource name out=w2324:refnum<visa-resource-name>)  [unwired: 1 in, 2 out]
                n1568 = Concatenate Strings("irun" ("string"), "\r") -> (w2331:string)
                n1569 = VISA Write(VISA resource name=w2324, write buffer=w2331) -> ()  [unwired: 1 in, 3 out]
              }
            }
            n1570 = local read "Saving..."() -> (w2300:bool)
            n1571 = local read "Save Event Log?"() -> (w2299:bool)
            n1572 = And(x=w2300, y=w2299) -> (x .and. y?=w2301:bool)
            n1573 = case shown="True" w2301 {
              tunnel: w2302 -> [_ w2313]
              frame False {
              }
              frame True {
                n1574 = local read "Normal Flow Rate (ul/h) P1"() -> (w2304:dbl)
                n1575 = Number To Decimal String(number=w2304) -> (decimal integer string=w2305:string)  [unwired: 1 in]
                n1576 = Concatenate Strings("on, flow rate", w2305) -> (w2307:string)
                n1577 = Select(t=w2307, s=w2313, f="off") -> (s? t:f=w2309:string)
                n1578 = local read "log file ref"() -> (w2314:refnum<file>)
                n1579 = local read "Time (s)"() -> (w2308:dbl)
                n1580 = Concatenate Strings("pump 1 ", w2309) -> (w2311:string)
                n1581 = call "write to event log.vi"("log file ref"=w2314, "time"=w2308, "input string"=w2311) -> ()  [unwired: 8 in]
              }
            }
          }
        }
      }
      event "Inject Pump 3": Value Change {
        n1582 = event-data() -> ()  [unwired: 7 out]
        n1583 = local read "Use Harvard pumps\nfor beads (else Chemyx)"() -> (w2334:bool)
        n1584 = case shown="True" w2334 {
          tunnel: "Inject Pump 3" -> [w2338 w2379]
          tunnel: w2333 -> [_ w2380]
          frame False {
            n1585 = local read "Pump write delay (ms)"() -> (w2337:dbl)
            n1586 = case shown="True" w2338 {
              tunnel: w2337 -> [w2344 w2358]
              tunnel: "Chemyx Syringe Pump Serial Port" -> [w2341 w2357]
              frame False {
                n1587 = flat-sequence {
                  tunnel: w2341 -> [w2345]
                  tunnel: [w2345] -> w2342
                  tunnel: w2344 -> [_]
                  tunnel: [w2348] -> w2343
                  tunnel: w2342 -> [w2348]
                  tunnel: w2343 -> [w2349]
                  tunnel: [w2349] -> w2339
                  tunnel: [w2351] -> w2340
                  tunnel: w2339 -> [w2351]
                  tunnel: w2340 -> [w2353]
                  frame #0 {
                    n1588 = call "Write to pump.vi"("string"="enter pump3", "VISA resource name"=w2345) -> ()  [unwired: 1 out]
                  }
                  frame #1 {
                    n1589 = local read "Pump pause delay (ms)"() -> (w2347:u32)
                    n1590 = Wait (ms)(milliseconds to wait=w2347) -> ()  [unwired: 1 out]
                  }
                  frame #2 {
                    n1591 = call "Write to pump.vi"("string"="stop", "VISA resource name"=w2349) -> ()  [unwired: 1 out]
                  }
                  frame #3 {
                    n1592 = Wait (ms)(milliseconds to wait=u32 0) -> ()  [unwired: 1 out]
                  }
                  frame #4 {
                    n1593 = call "Write to pump.vi"("string"="stop", "VISA resource name"=w2353) -> ()  [unwired: 1 out]
                  }
                }
              }
              frame True {
                n1594 = flat-sequence {
                  tunnel: w2357 -> [w2367]
                  tunnel: w2358 -> [w2362]
                  tunnel: w2358 -> [w2369]
                  tunnel: w2357 -> [w2370]
                  tunnel: [w2370] -> w2356
                  tunnel: [w2373] -> w2355
                  tunnel: w2356 -> [w2373]
                  tunnel: w2355 -> [w2374]
                  frame #0 {
                    n1595 = local read "All Pump Parameters"() -> (w2361:T7)
                    n1596 = Unbundle By Name(w2361) -> ("Pump 3"=w2368:T36)
                    n1597 = call "Set pump parameters.vi"("Pump write delay (ms)"=w2362, "Volume (uL)"="Ch 3 Inject Volume (uL)", "Rate (uL/h)"="Ch 3 Inject Rate (ul/h)", "Units"=4.0, "Pump #"=3.0, "Pump Parameters In"=w2368, "VISA resource name"=w2367) -> ("Pump Parameters Out"=w2360:T36)  [unwired: 3 in]
                    n1598 = Bundle By Name(cluster=w2361, "Pump 3"=w2360) -> (w2359:T7)
                    n1599 = local write "All Pump Parameters"(w2359) -> ()
                  }
                  frame #1 {
                    n1600 = Wait (ms)(milliseconds to wait=w2369) -> ()  [unwired: 1 out]
                  }
                  frame #2 {
                    n1601 = call "Write to pump.vi"("string"="start", "VISA resource name"=w2370) -> ()  [unwired: 1 out]
                  }
                  frame #3 {
                    n1602 = Wait (ms)(milliseconds to wait=u32 500) -> ()  [unwired: 1 out]
                  }
                  frame #4 {
                    n1603 = call "Write to pump.vi"("string"="start", "VISA resource name"=w2374) -> ()  [unwired: 1 out]
                  }
                }
              }
            }
          }
          frame True {
            n1604 = case shown="False" w2379 {
              tunnel: w2380 -> [w2392 w2399]
              frame False {
                n1605 = flat-sequence {
                  tunnel: w2392 -> [w2394]
                  frame #0 {
                    n1606 = local write "Flushing P3"(FALSE ("Flushing P3")) -> ()
                    n1607 = Concatenate Strings("stop" ("string"), "\r") -> (w2396:string)
                    n1608 = VISA Write(VISA resource name=w2394, write buffer=w2396) -> ()  [unwired: 1 in, 3 out]
                  }
                  frame #1 {
                    n1609 = property on="Clear Volume P3" class="Bool (strict)"("Val(Sgnl)"=TRUE ("Value (Signaling)")) -> ()  [unwired: 2 in, 2 out]
                  }
                }
              }
              frame True {
                n1610 = local read "Normal Flow Rate (ul/h) P3"() -> (w2400:dbl)
                n1611 = Number To Decimal String(number=w2400) -> (decimal integer string=w2406:string)  [unwired: 1 in]
                n1612 = Concatenate Strings("irate  " ("string"), w2406, " u/h" ("string"), "\r") -> (w2404:string)
                n1613 = VISA Write(VISA resource name=w2399, write buffer=w2404) -> (VISA resource name out=w2402:refnum<visa-resource-name>)  [unwired: 1 in, 2 out]
                n1614 = Concatenate Strings("irun" ("string"), "\r") -> (w2408:string)
                n1615 = VISA Write(VISA resource name=w2402, write buffer=w2408) -> ()  [unwired: 1 in, 3 out]
              }
            }
            n1616 = local read "Save Event Log?"() -> (w2377:bool)
            n1617 = local read "Saving..."() -> (w2378:bool)
            n1618 = And(x=w2378, y=w2377) -> (x .and. y?=w2376:bool)
            n1619 = case shown="True" w2376 {
              tunnel: w2379 -> [_ w2387]
              frame False {
              }
              frame True {
                n1620 = local read "Normal Flow Rate (ul/h) P3"() -> (w2381:dbl)
                n1621 = Number To Decimal String(number=w2381) -> (decimal integer string=w2383:string)  [unwired: 1 in]
                n1622 = Concatenate Strings("on, flow rate", w2383) -> (w2382:string)
                n1623 = local read "log file ref"() -> (w2386:refnum<file>)
                n1624 = Select(t=w2382, s=w2387, f="off") -> (s? t:f=w2388:string)
                n1625 = local read "Time (s)"() -> (w2385:dbl)
                n1626 = Concatenate Strings("pump 3 ", w2388) -> (w2390:string)
                n1627 = call "write to event log.vi"("log file ref"=w2386, "time"=w2385, "input string"=w2390) -> ()  [unwired: 8 in]
              }
            }
          }
        }
      }
      event "Inject Pump 2": Value Change {
        n1628 = event-data() -> ()  [unwired: 7 out]
        n1629 = local read "Pump write delay (ms)"() -> (w2415:dbl)
        n1630 = flat-sequence {
          tunnel: w2414 -> [w2439]
          tunnel: w2415 -> [w2435]
          tunnel: "Inject Pump 2" -> [_]
          tunnel: w2415 -> [w2441]
          tunnel: w2414 -> [w2442]
          frame #0 {
            n1631 = local read "All Pump Parameters"() -> (w2434:T7)
            n1632 = Multiply(x=60.0, y="Flush Center Ch Rate (ul/m)") -> (x*y=w2431:dbl)
            n1633 = Unbundle By Name(w2434) -> ("Pump 2"=w2440:T36)
            n1634 = call "Set pump parameters.vi"("Pump write delay (ms)"=w2435, "Volume (uL)"="Flush Center Ch Volume (uL)", "Rate (uL/h)"=w2431, "Units"=3.0, "Pump #"=2.0, "Pump Parameters In"=w2440, "VISA resource name"=w2439) -> ("Pump Parameters Out"=w2433:T36)  [unwired: 3 in]
            n1635 = Bundle By Name(cluster=w2434, "Pump 2"=w2433) -> (w2432:T7)
            n1636 = local write "All Pump Parameters"(w2432) -> ()
            n1637 = Add(x="Flush Center Ch Volume (uL)", y="Total Volume\nFlushed (uL)") -> (x+y=w2428:dbl)
            n1638 = local write "Total Volume\nFlushed (uL)"(w2428) -> ()
          }
          frame #1 {
            n1639 = Wait (ms)(milliseconds to wait=w2441) -> ()  [unwired: 1 out]
          }
          frame #2 {
            n1640 = call "Write to pump.vi"("string"="start", "VISA resource name"=w2442) -> ()  [unwired: 1 out]
          }
        }
        n1641 = local read "Chemyx Syringe Pump Serial Port"() -> (w2414:refnum<visa-resource-name>)
        n1642 = local read "Save Event Log?"() -> (w2413:bool)
        n1643 = local read "Saving..."() -> (w2412:bool)
        n1644 = And(x=w2413, y=w2412) -> (x .and. y?=w2411:bool)
        n1645 = case shown="True" w2411 {
          tunnel: "Inject Pump 2" -> [_ w2422]
          frame False {
          }
          frame True {
            n1646 = local read "Flow rate (uL/h)"() -> (w2416:dbl)
            n1647 = Number To Decimal String(number=w2416) -> (decimal integer string=w2418:string)  [unwired: 1 in]
            n1648 = Concatenate Strings("on, flow rate", w2418) -> (w2417:string)
            n1649 = Select(t=w2417, s=w2422, f="off") -> (s? t:f=w2426:string)
            n1650 = local read "Time (s)"() -> (w2420:dbl)
            n1651 = local read "log file ref"() -> (w2421:refnum<file>)
            n1652 = Concatenate Strings("pump 2 ", w2426) -> (w2424:string)
            n1653 = call "write to event log.vi"("log file ref"=w2421, "time"=w2420, "input string"=w2424) -> ()  [unwired: 8 in]
          }
        }
      }
      event "Sample Channel\nFlow": Value Change {
        n1654 = event-data() -> ()  [unwired: 7 out]
        n1655 = Select(t="irun" ("string"), s="Sample Channel\nFlow", f="stop" ("string")) -> (s? t:f=w2446:string)
        n1656 = Concatenate Strings(w2446, "\r") -> (w2449:string)
        n1657 = VISA Write(VISA resource name=w2444, write buffer=w2449) -> ()  [unwired: 1 in, 3 out]
      }
      event "Start Flow": Value Change {
        n1658 = event-data() -> ()  [unwired: 7 out]
        n1659 = local write "Sample Channel\nFlow"(TRUE ("Sample Channel\nFlow")) -> ()
        n1660 = local write "Start Flow"(FALSE ("Start Flow")) -> ()
        n1661 = Concatenate Strings("irun" ("string"), "\r") -> (w2455:string)
        n1662 = VISA Write(VISA resource name=w2451, write buffer=w2455) -> ()  [unwired: 1 in, 3 out]
      }
      event "Stop Flow": Value Change {
        w2457 = FALSE ("Stop Flow")
        n1663 = event-data() -> ()  [unwired: 7 out]
        n1664 = local write "Stop Flow"(w2457) -> ()
        n1665 = local write "Sample Channel\nFlow"(w2457) -> ()
        n1666 = Concatenate Strings("stop" ("string"), "\r") -> (w2460:string)
        n1667 = VISA Write(VISA resource name=w2458, write buffer=w2460) -> ()  [unwired: 1 in, 3 out]
      }
      event "Flow rate (uL/h)": Value Change {
        n1668 = event-data() -> ()  [unwired: 7 out]
        n1669 = Number To Decimal String(number="Flow rate (uL/h)") -> (decimal integer string=w2467:string)  [unwired: 1 in]
        n1670 = Concatenate Strings("irate  " ("string"), w2467, " u/h" ("string"), "\r") -> (w2466:string)
        n1671 = VISA Write(VISA resource name=w2463, write buffer=w2466) -> ()  [unwired: 1 in, 3 out]
      }
      event "Flush Sample": Value Change {
        n1672 = event-data() -> ()  [unwired: 7 out]
        n1673 = flat-sequence {
          tunnel: w2477 -> [w2515]
          tunnel: [w2495] -> w2476
          tunnel: [w2491] -> w2474
          tunnel: ["Volume (uL)"] -> w2473
          tunnel: ["Flush rate (uL/m)"] -> w2472
          tunnel: w2476 -> [w2519]
          tunnel: [w2519] -> w2475
          tunnel: w2474 -> [w2518]
          tunnel: w2475 -> [w2524]
          frame #0 {
            # "set paramaters (rate, volume) for flush, clear volume"
            n1674 = Number To Decimal String(number="Flush rate (uL/m)") -> (decimal integer string=w2511:string)  [unwired: 1 in]
            n1675 = Concatenate Strings("irate  " ("string"), w2511, " u/m" ("string"), "\r") -> (w2513:string)
            n1676 = VISA Write(VISA resource name=w2515, write buffer=w2513) -> (VISA resource name out=w2509:refnum<visa-resource-name>)  [unwired: 1 in, 2 out]
            n1677 = Reciprocal(x="Flush rate (uL/m)") -> (1/x=w2494:dbl)
            n1678 = Number To Decimal String(number="Volume (uL)") -> (decimal integer string=w2500:string)  [unwired: 1 in]
            n1679 = Multiply(x="Volume (uL)", y=w2494) -> (x*y=w2493:dbl)
            n1680 = Concatenate Strings("tvolume  " ("string"), w2500, " u" ("string"), "\r") -> (w2498:string)
            n1681 = Multiply(x=w2493, y=60000.0) -> (x*y=w2491:dbl)
            n1682 = VISA Write(VISA resource name=w2509, write buffer=w2498) -> (VISA resource name out=w2497:refnum<visa-resource-name>)  [unwired: 1 in, 2 out]
            n1683 = Concatenate Strings("cvolume" ("string"), "\r") -> (w2496:string)
            n1684 = VISA Write(VISA resource name=w2497, write buffer=w2496) -> (VISA resource name out=w2507:refnum<visa-resource-name>)  [unwired: 1 in, 2 out]
            n1685 = Concatenate Strings("irun" ("string"), "\r") -> (w2505:string)
            n1686 = VISA Write(VISA resource name=w2507, write buffer=w2505) -> (VISA resource name out=w2495:refnum<visa-resource-name>)  [unwired: 1 in, 2 out]
          }
          frame #1 {
            # "Have to wait until\nflow is done to reset\nrate"
            n1687 = Add(x=w2518, y=100.0) -> (x+y=w2517:dbl)
            n1688 = Wait (ms)(milliseconds to wait=w2517) -> ()  [unwired: 1 out]
          }
          frame #2 {
            # "reset flow rate to usual flow rate"
            n1689 = local read "Flow rate (uL/h)"() -> (w2530:dbl)
            n1690 = Number To Decimal String(number=w2530) -> (decimal integer string=w2528:string)  [unwired: 1 in]
            n1691 = Concatenate Strings("irate  " ("string"), w2528, " u/h" ("string"), "\r") -> (w2526:string)
            n1692 = VISA Write(VISA resource name=w2524, write buffer=w2526) -> (VISA resource name out=w2520:refnum<visa-resource-name>)  [unwired: 1 in, 2 out]
            n1693 = Concatenate Strings("cvolume" ("string"), "\r") -> (w2521:string)
            n1694 = VISA Write(VISA resource name=w2520, write buffer=w2521) -> ()  [unwired: 1 in, 3 out]
          }
        }
        n1695 = local read "Save Event Log?"() -> (w2470:bool)
        n1696 = local read "Saving..."() -> (w2469:bool)
        n1697 = And(x=w2470, y=w2469) -> (x .and. y?=w2471:bool)
        n1698 = case shown="True" w2471 {
          tunnel: w2473 -> [_ w2480]
          tunnel: w2472 -> [_ w2479]
          frame False {
          }
          frame True {
            n1699 = Number To Decimal String(number=w2480) -> (decimal integer string=w2484:string)  [unwired: 1 in]
            n1700 = Number To Decimal String(number=w2479) -> (decimal integer string=w2486:string)  [unwired: 1 in]
            n1701 = local read "log file ref"() -> (w2481:refnum<file>)
            n1702 = local read "Time (s)"() -> (w2482:dbl)
            n1703 = Concatenate Strings("pump 2 flushing ", w2484, " uL at ", w2486, " ul/min") -> (w2488:string)
            n1704 = call "write to event log.vi"("log file ref"=w2481, "time"=w2482, "input string"=w2488) -> ()  [unwired: 8 in]
          }
        }
      }
      event "Flush Pump 3": Value Change {
        n1705 = event-data() -> ()  [unwired: 7 out]
        n1706 = flat-sequence {
          tunnel: w2536 -> [w2551]
          tunnel: ["Flush rate (uL/m) P3"] -> w2532
          tunnel: ["Volume (uL) P3"] -> w2531
          frame #0 {
            # "set paramaters (rate, volume) for flush, clear volume"
            n1707 = Number To Decimal String(number="Flush rate (uL/m) P3") -> (decimal integer string=w2571:string)  [unwired: 1 in]
            n1708 = local write "Inject Pump 3"(TRUE ("Inject Pump 3")) -> ()
            n1709 = Concatenate Strings("irate  " ("string"), w2571, " u/m" ("string"), "\r") -> (w2573:string)
            n1710 = VISA Write(VISA resource name=w2551, write buffer=w2573) -> (VISA resource name out=w2569:refnum<visa-resource-name>)  [unwired: 1 in, 2 out]